vi "IMAQdx_AbsImage_Flea3_v4.6.vi"() -> ()   [LabVIEW 2013] (continued)
rMOTcurrF\trMOTpow3\tcombAmplitude(combWidthF)\trMOTdelta(-(rMOTbroadDetuningF +combWidthF/2))\tODTpowHLat(DipPowHLat2)\t0\t0\t0\t0\t0\t0\t1\t1\tbMOTdelta(MOTdetuning)\tbMOTpow(0.5)\tProbePow\tPdet2\tXshim\tYshim\tZshimVar\tODTpowZ(DipPowZLat)\t0\t1\t0\t0\t1\t0\t0\t0\t0\t0\t0\t0\t0\t0\t0\t0\t0\t0\trMOTdelta(-(rMOTstirDetI +stirWidthF/2))\tODTpowBlue(0)\tExpFinal(tEvap1,ODTpowXY(DipPowCr2),ODTpowXY(DipPowCr3),tau)\tvarWaveP2\tPdet\tAmp688(depumpPow)\trMOTpow3\tExpFinal(tEvap1,ODTpowX(DipPowX2),ODTpowX(DipPowX3),tau)\tfreq\tHeatingAmp\t0\tSine\tDetuning\tsingleFreqDet\tDoppCoolDet-DoppCoolSweep\tdopCoolT*1000\tDetuning\tsingleFreqStirDet + 20\tsingleFreqStirDet + 20\tSFcoolT*1000\tBlueBN\tBlueLaserProbeBN\tPixisPos(TOF)\tCycle Wait for Move\r\nlattice rampdown\t\tRamp\t0\trampLatOffT\t1\t1\t1\t1\t1\t1\t0\t0\t1\t1\t0\t0\t0\t1\t0\t0\t0\t1\t0\t0\t0\t0\t0\t0\t10u\t0\t1\t0\t0\t0\t1\t1\t0\tplus_zman\tminus_zman\tcompensation\trMOTcurrF\trMOTpow3\tcombAmplitude(combWidthF)\trMOTdelta(-(rMOTbroadDetuningF +combWidthF/2))\tSinRamp(t,(ODTpowHLat(DipPowHLat)+ODTpowHLat(DipPowHLat2))/2,(ODTpowHLat(DipPowHLat)-ODTpowHLat(DipPowHLat2))/2,1/(2*rampLatOffT), 3*pi/2)\t0\t0\t0\t0\t0\t0\t1\t1\tbMOTdelta(MOTdetuning)\tbMOTpow(0.5)\tProbePow\tPdet2\tXshim\tYshim\tZshimVar\tSinRamp(t,(ODTpowZ(DipPowZ3)+ODTpowZ(DipPowZLat))/2, (ODTpowZ(DipPowZ3)-ODTpowZ(DipPowZLat))/2, 1/(2*rampLatOffT), 3*pi/2)\t0\t1\t0\t0\t1\t0\t0\t0\t0\t0\t0\t0\t0\t0\t0\t0\t0\t0\trMOTdelta(-(rMOTstirDetI +stirWidthF/2))\tODTpowBlue(0)\tExpFinal(tEvap1,ODTpowXY(DipPowCr2),ODTpowXY(DipPowCr3),tau)\tLineRamp(f,varWaveP2,varWaveP1)\tPdet\tAmp688(depumpPow)\trMOTpow3\tExpFinal(tEvap1,ODTpowX(DipPowX2),ODTpowX(DipPowX3),tau)\tfreq\tHeatingAmp\t0\tSine\tDetuning\tsingleFreqDet\tDoppCoolDet-DoppCoolSweep\tdopCoolT*1000\tDetuning\tsingleFreqStirDet + 20\tsingleFreqStirDet + 20\tSFcoolT*1000\tBlueBN\tBlueLaserProbeBN\tPixisPos(TOF)\tCycle Wait for Move\r\nEvaporation\t\tRamp\t0\ttEvap2\t1\t1\t1\t1\t1\t1\t0\t0\t1\t1\t0\t0\t0\t1\t0\t0\t0\t1\t0\t0\t0\t0\t0\t0\t50u\t0\t1\t0\t0\t0\t1\t1\t0\tplus_zman\tminus_zman\tcompensation\trMOTcurrF\trMOTpow3\tcombAmplitude(combWidthF)\trMOTdelta(-(rMOTbroadDetuningF +combWidthF/2))\tODTpowHLat(DipPowHLat)\t0\t0\t0\t0\t0\t0\t1\t1\tbMOTdelta(MOTdetuning)\tbMOTpow(0.5)\tProbePow\tPdet2\tXshim\tYshim\tZshimVar\tLineRamp(f,ODTpowZ(DipPowZ3),ODTpowZ(DipPowZ4))\t0\t1\t0\t0\t0\t0\t0\t0\t0\t0\t0\t0\t0\t0\t0\t0\t0\t0\trMOTdelta(-(rMOTstirDetI +stirWidthF/2))\tODTpowBlue(0)\tExpRamp2(t,0,ExpFinal(tEvap1,ODTpowXY(DipPowCr2),ODTpowXY(DipPowCr3),tau),ODTpowXY(DipPowCr4),tau2)\tvarWaveP2\tPdet\tAmp688(depumpPow)\trMOTpow3\tExpRamp2(t,0,ExpFinal(tEvap1,ODTpowX(DipPowX2),ODTpowX(DipPowX3),tau),ODTpowX(DipPowX4),tau2)\tfreq\tHeatingAmp\t0\tSine\tDetuning\tsingleFreqDet\tDoppCoolDet-DoppCoolSweep\tdopCoolT*1000\tDetuning\tsingleFreqStirDet + 20\tsingleFreqStirDet + 20\tSFcoolT*1000\tBlueBN\tBlueLaserProbeBN\tPixisPos(TOF)\tCycle Wait for Move\r\npost evap hold\t\tRamp\t0\t.0075\t1\t1\t1\t1\t1\t1\t0\t0\t1\t1\t0\t0\t0\t1\t0\t0\t0\t1\t0\t0\t0\t0\t0\t0\t0\t0\t1\t0\t0\t0\t1\t1\t0\tplus_zman\tminus_zman\tcompensation\trMOTcurrF\trMOTpow3\tcombAmplitude(combWidthF)\trMOTdelta(-(rMOTbroadDetuningF +combWidthF/2))\tODTpowHLat(DipPowHLat)\t0\t0\t0\t0\t0\t0\t1\t1\tbMOTdelta(MOTdetuning)\tbMOTpow(0.5)\tProbePow\tPdet2\tXshim\tYshim\tZshimVar\tExpFinal(tEvap1,ODTpowZ(DipPowZ),ODTpowZ(DipPowZ2),tau)\tVimaging\t1\t0\t0\t0\t0\t0\t0\t0\t0\t0\t0\t0\t0\t0\t0\t0\t0\trMOTdelta(-(rMOTstirDetI +stirWidthF/2))\tODTpowBlue(0)\tExpFinal(tEvap1,ODTpowXY(DipPowCr),ODTpowXY(DipPowCr2),tau)\tvarWaveP2\tPdet\tAmp688(depumpPow)\trMOTpow3\tExpFinal(tEvap1,ODTpowX(DipPowX),ODTpowX(DipPowX2),tau)\tfreq\tHeatingAmp\t0\tSine\tDetuning\tsingleFreqDet\tDoppCoolDet-DoppCoolSweep\tdopCoolT*1000\tDetuning\tsingleFreqStirDet + 20\tsingleFreqStirDet + 20\tSFcoolT*1000\tBlueBN\tBlueLaserProbeBN\tPixisPos(TOF)\tCycle Wait for Move\r\nrMOT/Dip TOF\t\tRamp\t1\tTOFaux\t0\t0\t0\t0\t0\t0\t1\t0\t0\t1\t0\t0\t0\t0\t0\t0\t0\t1\t0\t0\t0\t0\t0\t0\t0\t0\t1\t0\t0\t0\t1\t1\t0\tplus_zman\tminus_zman\tcompensation\trMOTcurrF\trMOTpow5\tcombAmplitude(combWidthF)\trMOTdelta(-(rMOTbroadDetuningF +combWidthF/2))\tODTpowHLat(DipPowHLat2)\t0\tVimaging\t0\t0\t0\t1\t1\t1\tbMOTdelta(MOTdetuning)\tbMOTpow(0.5)\tProbePow\tPdet\tXshim\tYshim\tZshimVar\tODTpowZ(DipPowZ3)\tVimaging\t1\t0\tHimaging\t0\t0\t0\t0\t0\t0\t0\t0\t0\t0\t0\t0\t0\t0\trMOTdelta(-(rMOTstirDetI +stirWidthF/2))\tODTpowBlue(0)\tODTpowXY(DipPowCrTOF)\tvarWaveP2\tPdet\tAmp688(depumpPow)\trMOTpow6\tODTpowX(DipPowXTOF)\tfreq\tHeatingAmp\t0\tSine\tDetuning\tsingleFreqDetF\tDoppCoolDet-DoppCoolSweep\tdopCoolT*1000\tDetuning\tsingleFreqStirDet + 20\tsingleFreqStirDet + 20\tSFcoolT*1000\tBlueBN\tBlueLaserProbeBN\tPixisPos(TOF)\tCycle Wait for Move\r\nBEC in situ\t\tRamp\t0\tTOFaux\t1\t1\t1\t1\t1\t1\t1\t0\t0\t1\t0\t0\t0\t0\t0\t0\t0\t1\t0\t0\t0\t0\t0\t0\t0\t0\t1\t0\t0\t0\t1\t1\t0\tplus_zman\tminus_zman\tcompensation\trMOTcurrF\trMOTpow5\tcombAmplitude(combWidthF)\trMOTdelta(-(rMOTbroadDetuningF +combWidthF/2))\tODTpowHLat(DipPowHLat)\t0\tVimaging\t0\t0\t0\t1\t1\t1\tbMOTdelta(MOTdetuning)\tbMOTpow(0.5)\tProbePow\tPdet\tXshim\tYshim\tZshimVar\tODTpowZ(DipPowZ3)\tVimaging\t1\t0\tHimaging\t0\t0\t0\t0\t0\t0\t0\t0\t0\t0\t0\t0\t0\t0\trMOTdelta(-(rMOTstirDetI +stirWidthF/2))\tODTpowBlue(BlueDipPow)\tExpFinal(tEvap1,ODTpowXY(DipPowCr2),ODTpowXY(DipPowCr3),tau)\tvarWaveP1\tPdet\tAmp688(depumpPow)\trMOTpow6\tExpFinal(tEvap1,ODTpowX(DipPowX2),ODTpowX(DipPowX3),tau)\tfreq\tHeatingAmp\t0\tSine\tDetuning\tsingleFreqDetF\tDoppCoolDet-DoppCoolSweep\tdopCoolT*1000\tDetuning\tsingleFreqStirDet + 20\tsingleFreqStirDet + 20\tSFcoolT*1000\tBlueBN\tBlueLaserProbeBN\tPixisPos(TOF)\tCycle Wait for Move\r\nTOF\t\tRamp\t0\t.005\t0\t0\t0\t0\t0\t0\t1\t0\t0\t0\t0\t0\t0\t0\t0\t0\t0\t1\t0\t0\t0\t0\t0\t0\t0\t0\t1\t0\t0\t0\t1\t1\t0\tplus_zman\tminus_zman\tcompensation\trMOTcurrF\trMOTpow3\tcombAmplitude(combWidthF)\trMOTdelta(-(rMOTbroadDetuningF +combWidthF/2))\tODTpowHLat(DipPowHLat)\t1\tVimaging\t0\t0\t0\t1\t1\t1\tbMOTdelta(MOTdetuning)\tbMOTpow(0.5)\tProbePow\tPdet\tXshim\tYshim\tZshimVar\tODTpowZ(DipPowZ)\tVimaging\t1\t0\tHimaging\t0\t0\t0\t0\t0\t0\t0\t0\t0\t0\t0\t0\t0\t0\trMOTdelta(-(rMOTstirDetI +stirWidthF/2))\tODTpowBlue(0)\tODTpowXY(DipPowCr)\tvarWaveP2\tPdet\tAmp688(depumpPow)\trMOTpow3\tODTpowX(DipPowX2)\tfreq\tHeatingAmp\t0\tSine\tDetuning\tsingleFreqDet\tDoppCoolDet-DoppCoolSweep\tdopCoolT*1000\tDetuning\tsingleFreqStirDet\tsingleFreqStirDet + 20\tSFcoolT*1000\tBlueBN\tBlueLaserProbeBN\tPixisPos(TOF)\tCycle Wait for Move\r\nTOF\t\tRamp\t1-rMOTon\t.001\t0\t0\t0\t0\t0\t0\t1\t0\t0\t0\t0\t0\t0\t0\t0\t0\t0\t1\t0\t0\t0\t0\t0\t0\t0\t0\t1\t0\t0\t0\t1\t1\t0\tplus_zman\tminus_zman\tcompensation\trMOTcurrF\trMOTpow3\tcombAmplitude(combWidthF)\trMOTdelta(-(rMOTbroadDetuningF +combWidthF/2))\tODTpowHLat(DipPowHLat)\t1\tVimaging\t0\t0\t0\t1\t1\t1\tbMOTdelta(MOTdetuning)\tbMOTpow(0.5)\tProbePow\tPdet\tXshim\tYshim\tZshimVar\tODTpowZ(DipPowZ)\tVimaging\t1\t0\tHimaging\t0\t0\t0\t0\t0\t0\t0\t0\t0\t0\t0\t0\t0\t0\trMOTdelta(-(rMOTstirDetI +stirWidthF/2))\tODTpowBlue(0)\tODTpowXY(DipPowCr)\tvarWaveP2\tPdet\tAmp688(depumpPow)\trMOTpow3\tODTpowX(DipPowX2)\tfreq\tHeatingAmp\t0\tSine\tDetuning\tsingleFreqDet\tDoppCoolDet-DoppCoolSweep\tdopCoolT*1000\tDetuning\tsingleFreqStirDet\tsingleFreqStirDet + 20\tSFcoolT*1000\tBlueBN\tBlueLaserProbeBN\tPixisPos(TOF)\tCycle Wait for Move\r\narm DIP FLEA\t\tRamp\t1\tcameraArmT\t0\t0\t0\t0\t0\t0\t1\t0\t0\t0\t0\t0\t0\t0\t0\t0\t0\t0\t0\t0\t0\t0\t0\t0\t0\t0\t1\t0\t0\t0\t1\t0\t0\tplus_zman\tminus_zman\tcompensation\trMOTcurrF\trMOTpow3\tcombAmplitude(combWidthF)\trMOTdelta(-(rMOTbroadDetuningF +combWidthF/2))\tODTpowHLat(DipPowHLat)\t1\tVimaging\t0\t0\t0\t1\t1\t0\tbMOTdelta(MOTdetuning)\tbMOTpow(0.5)\tProbePow\tPdet\tXshim\tYshim\tZshimVar\tODTpowZ(DipPowZ3)\tVimaging\t1\t0\tHimaging\t0\t0\t0\t0\t0\t0\t0\t0\t0\t0\t0\t0\t0\t0\trMOTdelta(-(rMOTstirDetI +stirWidthF/2))\tODTpowBlue(0)\tODTpowXY(DipPowCrTOF)\tvarWaveP1\tPdet\tAmp688(depumpPow)\trMOTpow3\tODTpowX(DipPowXTOF)\tfreq\tHeatingAmp\t0\tSine\tDetuning\tsingleFreqDet\tDoppCoolDet-DoppCoolSweep\tdopCoolT*1000\tDetuning\tsingleFreqStirDet\tsingleFreqStirDet + 20\tSFcoolT*1000\tBlueBN\tBlueLaserProbeBN\tPixisPos(TOF)\tCycle Wait for Move\r\narm BEC FLEA\t\tRamp\t0\tcameraArmT\t0\t0\t0\t0\t0\t0\t1\t0\t0\t0\t0\t0\t0\t0\t0\t0\t0\t0\t0\t0\t0\t0\t0\t0\t0\t0\t1\t0\t0\t0\t1\t0\t0\tplus_zman\tminus_zman\tcompensation\trMOTcurrF\trMOTpow3\tcombAmplitude(combWidthF)\trMOTdelta(-(rMOTbroadDetuningF +combWidthF/2))\tODTpowHLat(DipPowHLat)\t1\tVimaging\t0\t0\t0\t1\t1\t0\tbMOTdelta(MOTdetuning)\tbMOTpow(0.5)\tProbePow\tPdet\tXshim\tYshim\tZshimVar\tODTpowZ(DipPowZ3)\tVimaging\t1\t0\tHimaging\t0\t0\t0\t0\t0\t0\t0\t0\t0\t0\t0\t0\t0\t0\trMOTdelta(-(rMOTstirDetI +stirWidthF/2))\tODTpowBlue(BlueDipPow)\tExpFinal(tEvap1,ODTpowXY(DipPowCr2),ODTpowXY(DipPowCr3),tau)\tvarWaveP1\tPdet\tAmp688(depumpPow)\trMOTpow3\tExpFinal(tEvap1,ODTpowX(DipPowX2),ODTpowX(DipPowX3),tau)\tfreq\tHeatingAmp\t0\tSine\tDetuning\tsingleFreqDet\tDoppCoolDet-DoppCoolSweep\tdopCoolT*1000\tDetuning\tsingleFreqStirDet\tsingleFreqStirDet + 20\tSFcoolT*1000\tBlueBN\tBlueLaserProbeBN\tPixisPos(TOF)\tCycle Wait for Move\r\natom img\t\tRamp\t1\texposureT\t0\t0\t0\t0\t0\t0\t1\t0\t1\t0\t0\t0\t0\t1\t0\t0\t0\t0\t0\t0\t0\t0\t0\t0\t0\t0\t1\t0\t0\t0\t1\t0\t0\tplus_zman\tminus_zman\tcompensation\trMOTcurrF\trMOTpow3\tcombAmplitude(combWidthF)\trMOTdelta(-(rMOTbroadDetuningF +combWidthF/2))\tODTpowHLat(DipPowHLat)\t1\tVimaging\t0\t0\t0\t1\t0\t0\tbMOTdelta(MOTdetuning)\tbMOTpow(0.5)\tProbePow\tPdet\tXshim\tYshim\tZshimVar\tODTpowZ(DipPowZ)\tVimaging\t1\t0\tHimaging\t0\t0\t0\t0\t0\t0\t0\t0\t0\t0\t0\t0\t0\t0\trMOTdelta(-(rMOTstirDetI +stirWidthF/2))\tODTpowBlue(0)\tODTpowXY(DipPowCr)\tvarWaveP1\tPdet\tAmp688(depumpPow)\trMOTpow3\tODTpowX(DipPowX)\tfreq\tHeatingAmp\t0\tSine\tDetuning\tsingleFreqDet\tDoppCoolDet-DoppCoolSweep\tdopCoolT*1000\tDetuning\tsingleFreqStirDet\tsingleFreqStirDet + 20\tSFcoolT*1000\tBlueBN\tBlueLaserProbeBN\tPixisPos(TOF)\tCycle Wait for Move\r\natom img\t\tRamp\t0\t2.8e-3\t0\t0\t0\t0\t0\t0\t1\t0\t0\t1\t0\t0\t0\t0\t0\t0\t0\t0\t0\t0\t0\t0\t0\t0\t0\t0\t1\t0\t0\t0\t1\t1\t0\tplus_zman\tminus_zman\tcompensation\trMOTcurrF\trMOTpow3\tcombAmplitude(combWidthF)\trMOTdelta(-(rMOTbroadDetuningF +combWidthF/2))\tODTpowHLat(DipPowHLat)\t1\tVimaging\t0\t0\t0\t1\t1\t1\tbMOTdelta(MOTdetuning)\tbMOTpow(0.5)\tProbePow\tPdet\tXshim\tYshim\tZshimVar\tODTpowZ(DipPowZ)\tVimaging\t1\t0\tHimaging\t0\t0\t0\t0\t0\t0\t0\t0\t0\t0\t0\t0\t0\t0\trMOTdelta(-(rMOTstirDetI +stirWidthF/2))\tODTpowBlue(0)\tODTpowXY(DipPowCr)\tvarWaveP2\tPdet\tAmp688(depumpPow)\trMOTpow3\tODTpowX(DipPowX)\tfreq\tHeatingAmp\t0\tSine\tDetuning\tsingleFreqDet\tDoppCoolDet-DoppCoolSweep\tdopCoolT*1000\tDetuning\tsingleFreqStirDet\tsingleFreqStirDet + 20\tSFcoolT*1000\tBlueBN\tBlueLaserProbeBN\tPixisPos(TOF)\tCycle Wait for Move\r\ntransmit img\t\tRamp\t1\t.625\t0\t0\t0\t0\t0\t0\t1\t0\t0\t1\t0\t0\t0\t0\t0\t0\t0\t0\t0\t0\t0\t0\t0\t0\t0\t0\t1\t0\t0\t0\t1\t1\t0\tplus_zman\tminus_zman\tcompensation\trMOTcurrF\trMOTpow3\tcombAmplitude(combWidthF)\trMOTdelta(-(rMOTbroadDetuningF +combWidthF/2))\tODTpowHLat(DipPowHLat)\t1\tVimaging\t0\t0\t0\t1\t1\t1\tbMOTdelta(MOTdetuning)\tbMOTpow(0.5)\tProbePow\tPdet\tXshim\tYshim\tZshimVar\tODTpowZ(DipPowZ)\tVimaging\t1\t0\tHimaging\t0\t0\t0\t0\t0\t0\t0\t0\t0\t0\t0\t0\t0\t0\trMOTdelta(-(rMOTstirDetI +stirWidthF/2))\tODTpowBlue(0)\tODTpowXY(DipPowCr)\tvarWaveP2\tPdet\tAmp688(depumpPow)\trMOTpow3\tODTpowX(DipPowX)\tfreq\tHeatingAmp\t0\tSine\tDetuning\tsingleFreqDet\tDoppCoolDet-DoppCoolSweep\tdopCoolT*1000\tDetuning\tsingleFreqStirDet\tsingleFreqStirDet + 20\tSFcoolT*1000\tBlueBN\tBlueLaserProbeBN\tPixisPos(TOF)\tCycle Wait for Move\r\narm PIXIS\t\tRamp\t0\t.007\t0\t0\t0\t0\t0\t0\t1\t0\t0\t1\t1\t0\t0\t0\t1\t1\t0\t0\t0\t0\t0\t0\t0\t0\t0\t0\t1\t0\t0\t0\t1\t1\t0\tplus_zman\tminus_zman\tcompensation\trMOTcurrF\trMOTpow1\tcombAmplitude(combWidthF)\trMOTdelta(-(rMOTbroadDetuningF +combWidthF/2))\tODTpowHLat(DipPowHLat)\t1\tVimaging\t0\t0\t0\t1\t1\t1\tbMOTdelta(MOTdetuning)\tbMOTpow(0.5)\tProbePow\tPdet\tXshim\tYshim\tZshimVar\tODTpowZ(DipPowZ)\tVimaging\t1\t0\tHimaging\t0\t0\t0\t0\t0\t0\t0\t0\t0\t0\t0\t0\t0\t0\trMOTdelta(-(rMOTstirDetI +stirWidthF/2))\tODTpowBlue(0)\tODTpowXY(DipPowCr)\tvarWaveP2\tPdet\tAmp688(depumpPow)\trMOTpow1\tODTpowX(DipPowX)\tfreq\tHeatingAmp\t0\tSine\tDetuning\tsingleFreqDet\tDoppCoolDet-DoppCoolSweep\tdopCoolT*1000\tDetuning\tsingleFreqStirDet\tsingleFreqStirDet + 20\tSFcoolT*1000\tBlueBN\tBlueLaserProbeBN\tPixisPos(TOF)\tCycle Wait for Move\r\narm FLEA\t\tRamp\t1\tcameraArmT\t0\t0\t0\t0\t0\t0\t1\t0\t0\t1\t1\t0\t0\t0\t1\t1\t0\t0\t0\t0\t0\t0\t0\t0\t0\t0\t1\t0\t0\t0\t1\t0\t0\tplus_zman\tminus_zman\tcompensation\trMOTcurrF\trMOTpow1\tcombAmplitude(combWidthF)\trMOTdelta(-(rMOTbroadDetuningF +combWidthF/2))\tODTpowHLat(DipPowHLat)\t1\tVimaging\t0\t0\t0\t1\t1\t0\tbMOTdelta(MOTdetuning)\tbMOTpow(0.5)\tProbePow\tPdet\tXshim\tYshim\tZshimVar\tODTpowZ(DipPowZ)\tVimaging\t1\t0\tHimaging\t0\t0\t0\t0\t0\t0\t0\t0\t0\t0\t0\t0\t0\t0\trMOTdelta(-(rMOTstirDetI +stirWidthF/2))\tODTpowBlue(0)\tODTpowXY(DipPowCr)\tvarWaveP2\tPdet\tAmp688(depumpPow)\trMOTpow1\tODTpowX(DipPowX)\tfreq\tHeatingAmp\t0\tSine\tDetuning\tsingleFreqDet\tDoppCoolDet-DoppCoolSweep\tdopCoolT*1000\tDetuning\tsingleFreqStirDet\tsingleFreqStirDet + 20\tSFcoolT*1000\tBlueBN\tBlueLaserProbeBN\tPixisPos(TOF)\tCycle Wait for Move\r\nprobe img\t\tRamp\t1\texposureT\t0\t0\t0\t0\t0\t0\t1\t0\t1\t1\t1\t0\t0\t1\t1\t1\t0\t0\t0\t0\t0\t0\t0\t0\t0\t0\t1\t0\t0\t0\t1\t0\t0\tplus_zman\tminus_zman\tcompensation\trMOTcurrF\trMOTpow1\tcombAmplitude(combWidthF)\trMOTdelta(-(rMOTbroadDetuningF +combWidthF/2))\tODTpowHLat(DipPowHLat)\t1\tVimaging\t0\t0\t0\t1\t0\t0\tbMOTdelta(MOTdetuning)\tbMOTpow(0.5)\tProbePow\tPdet\tXshim\tYshim\tZshimVar\tODTpowZ(DipPowZ)\tVimaging\t1\t0\tHimaging\t0\t0\t0\t0\t0\t0\t0\t0\t0\t0\t0\t0\t0\t0\trMOTdelta(-(rMOTstirDetI +stirWidthF/2))\tODTpowBlue(0)\tODTpowXY(DipPowCr)\tvarWaveP2\tPdet\tAmp688(depumpPow)\trMOTpow1\tODTpowX(DipPowX)\tfreq\tHeatingAmp\t0\tSine\tDetuning\tsingleFreqDet\tDoppCoolDet-DoppCoolSweep\tdopCoolT*1000\tDetuning\tsingleFreqStirDet\tsingleFreqStirDet + 20\tSFcoolT*1000\tBlueBN\tBlueLaserProbeBN\tPixisPos(TOF)\tCycle Wait for Move\r\nprobe img\t\tRamp\t0\t2.8e-3\t0\t0\t0\t0\t0\t0\t1\t0\t0\t1\t1\t0\t0\t0\t1\t1\t0\t0\t0\t0\t0\t0\t0\t0\t0\t0\t1\t0\t0\t0\t1\t1\t0\tplus_zman\tminus_zman\tcompensation\trMOTcurrF\trMOTpow1\tcombAmplitude(combWidthF)\trMOTdelta(-(rMOTbroadDetuningF +combWidthF/2))\tODTpowHLat(DipPowHLat)\t1\tVimaging\t0\t0\t0\t1\t1\t1\tbMOTdelta(MOTdetuning)\tbMOTpow(0.5)\tProbePow\tPdet\tXshim\tYshim\tZshimVar\tODTpowZ(DipPowZ)\tVimaging\t1\t0\tHimaging\t0\t0\t0\t0\t0\t0\t0\t0\t0\t0\t0\t0\t0\t0\trMOTdelta(-(rMOTstirDetI +stirWidthF/2))\tODTpowBlue(0)\tODTpowXY(DipPowCr)\tvarWaveP2\tPdet\tAmp688(depumpPow)\trMOTpow1\tODTpowX(DipPowX)\tfreq\tHeatingAmp\t0\tSine\tDetuning\tsingleFreqDet\tDoppCoolDet-DoppCoolSweep\tdopCoolT*1000\tDetuning\tsingleFreqStirDet\tsingleFreqStirDet + 20\tSFcoolT*1000\tBlueBN\tBlueLaserProbeBN\tPixisPos(TOF)\tCycle Wait for Move\r\ntransmit img\t\tRamp\t1\t.610\t0\t0\t0\t0\t0\t0\t1\t0\t0\t1\t1\t0\t0\t0\t1\t1\t0\t0\t0\t0\t0\t0\t0\t0\t0\t0\t1\t0\t0\t0\t1\t1\t0\tplus_zman\tminus_zman\tcompensation\trMOTcurrF\trMOTpow1\tcombAmplitude(combWidthF)\trMOTdelta(-(rMOTbroadDetuningF +combWidthF/2))\tODTpowHLat(DipPowHLat)\t1\tVimaging\t0\t0\t0\t1\t1\t1\tbMOTdelta(MOTdetuning)\tbMOTpow(0.5)\tProbePow\tPdet\tXshim\tYshim\tZshimVar\tODTpowZ(DipPowZ)\tVimaging\t1\t0\tHimaging\t0\t0\t0\t0\t0\t0\t0\t0\t0\t0\t0\t0\t0\t0\trMOTdelta(-(rMOTstirDetI +stirWidthF/2))\tODTpowBlue(0)\tODTpowXY(DipPowCr)\tvarWaveP2\tPdet\tAmp688(depumpPow)\trMOTpow1\tODTpowX(DipPowX)\tfreq\tHeatingAmp\t0\tSine\tDetuning\tsingleFreqDet\tDoppCoolDet-DoppCoolSweep\tdopCoolT*1000\tDetuning\tsingleFreqStirDet\tsingleFreqStirDet + 20\tSFcoolT*1000\tBlueBN\tBlueLaserProbeBN\tPixisPos(TOF)\tCycle Wait for Move\r\ntransmit img\t\tRamp\t1\t.015\t0\t0\t0\t0\t0\t0\t1\t0\t0\t1\t1\t0\t0\t0\t1\t1\t0\t0\t0\t0\t0\t0\t0\t0\t0\t0\t1\t0\t0\t0\t1\t1\t0\tplus_zman\tminus_zman\tcompensation\trMOTcurrF\trMOTpow1\tcombAmplitude(combWidthF)\trMOTdelta(-(rMOTbroadDetuningF +combWidthF/2))\tODTpowHLat(DipPowHLat2)\t1\tVimaging\t0\t0\t0\t1\t1\t1\tbMOTdelta(MOTdetuning)\tbMOTpow(0.5)\tProbePow\tPdet\tXshim\tYshim\tZshimVar\tODTpowZ(DipPowZ)\tVimaging\t1\t0\tHimaging\t0\t0\t0\t0\t0\t0\t0\t0\t0\t0\t0\t0\t0\t0\trMOTdelta(-(rMOTstirDetI +stirWidthF/2))\tODTpowBlue(.05)\tODTpowXY(DipPowCr)\tvarWaveP2\tPdet\tAmp688(depumpPow)\trMOTpow1\tODTpowX(DipPowX)\tfreq\tHeatingAmp\t0\tSine\tDetuning\tsingleFreqDet\tDoppCoolDet-DoppCoolSweep\tdopCoolT*1000\tDetuning\tsingleFreqStirDet\tsingleFreqStirDet + 20\tSFcoolT*1000\tBlueBN\tBlueLaserProbeBN\tPixisPos(TOF)\tCycle Wait for Move\r\narm PIXIS\t\tRamp\t0\t.007\t0\t0\t0\t0\t0\t0\t1\t0\t0\t1\t1\t0\t0\t0\t1\t1\t0\t0\t0\t0\t0\t0\t0\t0\t0\t0\t1\t0\t0\t0\t1\t0\t0\tplus_zman\tminus_zman\tcompensation\trMOTcurrF\trMOTpow1\tcombAmplitude(combWidthF)\trMOTdelta(-(rMOTbroadDetuningF +combWidthF/2))\tODTpowHLat(DipPowHLat2)\t1\tVimaging\t0\t0\t0\t1\t1\t1\tbMOTdelta(MOTdetuning)\tbMOTpow(0.5)\tProbePow\tPdet\tXshim\tYshim\tZshimVar\tODTpowZ(DipPowZ)\tVimaging\t1\t0\tHimaging\t0\t0\t0\t0\t0\t0\t0\t0\t0\t0\t0\t0\t0\t0\trMOTdelta(-(rMOTstirDetI +stirWidthF/2))\tODTpowBlue(0)\tODTpowXY(DipPowCr)\tvarWaveP2\tPdet\tAmp688(depumpPow)\trMOTpow1\tODTpowX(DipPowX)\tfreq\tHeatingAmp\t0\tSine\tDetuning\tsingleFreqDet\tDoppCoolDet-DoppCoolSweep\tdopCoolT*1000\tDetuning\tsingleFreqStirDet\tsingleFreqStirDet + 20\tSFcoolT*1000\tBlueBN\tBlueLaserProbeBN\tPixisPos(TOF)\tCycle Wait for Move\r\narm FLEA\t\tRamp\t1\tcameraArmT\t0\t0\t0\t0\t0\t0\t1\t0\t0\t1\t1\t0\t0\t0\t1\t1\t0\t0\t0\t0\t0\t0\t0\t0\t0\t0\t1\t0\t0\t0\t1\t0\t0\tplus_zman\tminus_zman\tcompensation\trMOTcurrF\trMOTpow1\tcombAmplitude(combWidthF)\trMOTdelta(-(rMOTbroadDetuningF +combWidthF/2))\tODTpowHLat(DipPowHLat2)\t1\tVimaging\t0\t0\t0\t1\t1\t0\tbMOTdelta(MOTdetuning)\tbMOTpow(0.5)\tProbePow\tPdet\tXshim\tYshim\tZshimVar\tODTpowZ(DipPowZ)\tVimaging\t1\t0\tHimaging\t0\t0\t0\t0\t0\t0\t0\t0\t0\t0\t0\t0\t0\t0\trMOTdelta(-(rMOTstirDetI +stirWidthF/2))\tODTpowBlue(.05)\tODTpowXY(DipPowCr)\tvarWaveP2\tPdet\tAmp688(depumpPow)\trMOTpow1\tODTpowX(DipPowX)\tfreq\tHeatingAmp\t0\tSine\tDetuning\tsingleFreqDet\tDoppCoolDet-DoppCoolSweep\tdopCoolT*1000\tDetuning\tsingleFreqStirDet\tsingleFreqStirDet + 20\tSFcoolT*1000\tBlueBN\tBlueLaserProbeBN\tPixisPos(TOF)\tCycle Wait for Move\r\nbg img\t\tRamp\t1\texposureT\t0\t0\t0\t0\t0\t0\t1\t0\t0\t1\t1\t0\t0\t0\t1\t1\t0\t0\t0\t0\t0\t0\t0\t0\t0\t0\t1\t0\t0\t0\t1\t0\t0\tplus_zman\tminus_zman\tcompensation\trMOTcurrF\trMOTpow1\tcombAmplitude(combWidthF)\trMOTdelta(-(rMOTbroadDetuningF +combWidthF/2))\tODTpowHLat(DipPowHLat2)\t1\tVimaging\t0\t0\t0\t1\t0\t0\tbMOTdelta(MOTdetuning)\tbMOTpow(0.5)\tProbePow\tPdet\tXshim\tYshim\tZshimVar\tODTpowZ(DipPowZ)\tVimaging\t1\t0\tHimaging\t0\t0\t0\t0\t0\t0\t0\t0\t0\t0\t0\t0\t0\t0\trMOTdelta(-(rMOTstirDetI +stirWidthF/2))\tODTpowBlue(0)\tODTpowXY(DipPowCr)\tvarWaveP2\tPdet\tAmp688(depumpPow)\trMOTpow1\tODTpowX(DipPowX)\tfreq\tHeatingAmp\t0\tSine\tDetuning\tsingleFreqDet\tDoppCoolDet-DoppCoolSweep\tdopCoolT*1000\tDetuning\tsingleFreqStirDet\tsingleFreqStirDet + 20\tSFcoolT*1000\tBlueBN\tBlueLaserProbeBN\tPixisPos(TOF)\tCycle Wait for Move\r\nbg img\t\tRamp\t0\t1e-4\t0\t0\t0\t0\t0\t0\t1\t0\t0\t1\t1\t0\t0\t0\t1\t1\t0\t0\t0\t0\t0\t0\t0\t0\t0\t0\t1\t0\t0\t0\t1\t1\t0\tplus_zman\tminus_zman\tcompensation\trMOTcurrF\trMOTpow1\tcombAmplitude(combWidthF)\trMOTdelta(-(rMOTbroadDetuningF +combWidthF/2))\tODTpowHLat(DipPowHLat)\t1\tVimaging\t0\t0\t0\t1\t1\t1\tbMOTdelta(MOTdetuning)\tbMOTpow(0.5)\tProbePow\tPdet\tXshim\tYshim\tZshimVar\tODTpowZ(DipPowZ)\tVimaging\t1\t0\tHimaging\t0\t0\t0\t0\t0\t0\t0\t0\t0\t0\t0\t0\t0\t0\trMOTdelta(-(rMOTstirDetI +stirWidthF/2))\tODTpowBlue(0)\tODTpowXY(DipPowCr)\tvarWaveP2\tPdet\tAmp688(depumpPow)\trMOTpow1\tODTpowX(DipPowX)\tfreq\tHeatingAmp\t0\tSine\tDetuning\tsingleFreqDet\tDoppCoolDet-DoppCoolSweep\tdopCoolT*1000\tDetuning\tsingleFreqStirDet\tsingleFreqStirDet + 20\tSFcoolT*1000\tBlueBN\tBlueLaserProbeBN\tPixisPos(TOF)\tCycle Wait for Move\r\ntransmit img\t\tRamp\t1\t.625\t0\t0\t0\t0\t0\t0\t1\t1\t0\t1\t1\t0\t0\t0\t1\t1\t0\t0\t0\t0\t0\t0\t0\t0\t0\t0\t1\t0\t0\t0\t1\t1\t0\tplus_zman\tminus_zman\tcompensation\trMOTcurrF\trMOTpow1\tcombAmplitude(combWidthF)\trMOTdelta(-(rMOTbroadDetuningF +combWidthF/2))\tODTpowHLat(DipPowHLat)\t1\tVimaging\t0\t0\t0\t1\t1\t1\tbMOTdelta(MOTdetuning)\tbMOTpow(0.5)\tProbePow\tLineRamp(f,Pdet,Pdet2)\tXshim\tYshim\tZshimVar\tODTpowZ(DipPowZ)\tVimaging\t1\t0\tHimaging\t0\t0\t0\t0\t0\t0\t0\t0\t0\t0\t0\t0\t0\t0\trMOTdelta(-(rMOTstirDetI +stirWidthF/2))\tODTpowBlue(0)\tODTpowXY(DipPowCr)\tvarWaveP2\tPdet\tAmp688(depumpPow)\trMOTpow1\tODTpowX(DipPowX)\tfreq\tHeatingAmp\t0\tSine\tDetuning\tsingleFreqDet\tDoppCoolDet-DoppCoolSweep\tdopCoolT*1000\tDetuning\tsingleFreqStirDet\tsingleFreqStirDet + 20\tSFcoolT*1000\tBlueBN\tBlueLaserProbeBN\tPixisPos(TOF)\tCycle Wait for Move\r\nalignment\t\tRamp\t1\t.1\t1\t1\t1\t1\t1\t1\t1\t0\t1\t0\t1\t0\t1\t1\t1\t1\t0\t0\t0\t0\t0\t0\t0\t0\t1m\t0\t1\t0\t1\t0\t0\t1\t1\tplus_zman\tminus_zman\tcompensation\tMOTcurrent\trMOTpow1\tcombAmplitude(combWidthI)\trMOTdelta(-(rMOTbroadDetuningI +combWidthI/2))\tODTpowHLat(DipPowHLat2)\t1\t0\t1\t1\t0\t1\t1\t1\tbMOTdelta(MOTdetuning)\tbMOTpow(MOTPow)\tProbePow\tPdet2\tXshim\tYshim\tZshim\tODTpowZ(DipPowZLat)\t0\t1\t0\t0\t0\t1\t0\t0\t0\t0\t0\t0\t0\t0\t0\t0\t0\t0\trMOTdelta(-(rMOTstirDetI +stirWidthI/2))\tODTpowBlue(0)\tODTpowXY(DipPowCr)\tvarWaveP2\tLineRamp(f,Pdet,BlueLaserLockOffset)\tAmp688(depumpPow)\trMOTpow3\tODTpowX(DipPowX)\tfreq\tHeatingAmp\t0\tSine\tRamp\tsingleFreqDet\tsingleFreqDetF\tSFcoolT*1000\tRamp\tsingleFreqStirDet\tsingleFreqStirDetF\tSFcoolT*1000\tBlueBN\tBlueLaserBeatnote\tPixisPos(TOF)\tCycle Wait for Move\r\n\r\n\r\n"
  in  "Flea Wave Name":string="Test_Img"
  in  "Save files to archive?":bool=TRUE
  out "Timeout":bool=TRUE
  out "Trigger Overrun":bool=TRUE
  in  "Source of File Data":refnum<k21>="\\\\Control\\VariableLibrary\\Instruction String"
  in  "Timeout (ms)":u32=20000
  in  "Gain":dbl
  in  "Shutter speed":dbl=30000.0
  in  "PIXIS Magnification":dbl=5.48
  in  "PIXIS Image direction":enum16{"XY", "XZ"}(ring)
  in  "PIXIS Imaging technique":enum16{"Absorption", "Fluorescence", "RawImage"}(ring)
  in  "SPE File Path":path=path "C:/Users/Lab/Documents/LightField/LabviewTemp.spe"
  in  "Send PIXIS data to Igor?":bool
  in  "PIXIS File Parameters":T1={"Data Root"=path "I:/Data", "Index"=4, "Instrument"="PIXIS"} {"Index" format="%04d"}
  in  "Source of Wavemeter Data":refnum<k21>="\\\\WS7PC\\VariableLibrary\\Frequency"
  in  "Accept wavelength from remote system":bool=TRUE
  in  "Flea Raw image to view":u16(ring)=1 items=["Clear", "Absorbtion", "Probe", "Background"]
  in  "Update Graphics":bool=TRUE
  out "Flea Raw Image":u16[][](graph)
  out "Flea Processed Image":sgl[][](graph)
  out "PIXIS Processed Image":sgl[][](graph)
  out "PIXIS Raw Image":u16[][](graph)
  in  "PIXIS Raw image to view":u16(ring)=1 items=["Clear", "Absorbtion", "Probe", "Background"]
  out "Camera Error":errorcluster={"status"=FALSE, "code"=-1074360293, "source"="IMAQdx Get Image2.vi"}
  out "DDE Error":errorcluster={"status"=FALSE, "code"=0, "source"="DDE Close: No Error"}
  out "Status Array":T4(array[cluster])=[{"AcquisitionInProgress"=FALSE, "BufferCount"=0, "LastBufferNumber"=4294967292, "LostBufferCount"=0}, {"AcquisitionInProgress"=TRUE, "BufferCount"=0, "LastBufferNumber"=4294967292, "LostBufferCount"=0}, {"AcquisitionInProgress"=TRUE, "BufferCount"=0, "LastBufferNumber"=4294967292, "LostBufferCount"=0}, {"AcquisitionInProgress"=TRUE, "BufferCount"=0, "LastBufferNumber"=4294967292, "LostBufferCount"=0}, {"AcquisitionInProgress"=TRUE, "BufferCount"=0, "LastBufferNumber"=4294967292, "LostBufferCount"=0}, {"AcquisitionInProgress"=TRUE, "BufferCount"=0, "LastBufferNumber"=4294967292, "LostBufferCount"=0}, {"AcquisitionInProgress"=TRUE, "BufferCount"=0, "LastBufferNumber"=4294967292, "LostBufferCount"=0}, {"AcquisitionInProgress"=TRUE, "BufferCount"=0, "LastBufferNumber"=4294967292, "LostBufferCount"=0}, {"AcquisitionInProgress"=TRUE, "BufferCount"=0, "LastBufferNumber"=4294967292, "LostBufferCount"=0}, {"AcquisitionInProgress"=TRUE, "BufferCount"=1, "LastBufferNumber"=0, "LostBufferCount"=0}, {"AcquisitionInProgress"=TRUE, "BufferCount"=2, "LastBufferNumber"=1, "LostBufferCount"=0}, {"AcquisitionInProgress"=TRUE, "BufferCount"=3, "LastBufferNumber"=2, "LostBufferCount"=0}, {"AcquisitionInProgress"=TRUE, "BufferCount"=4, "LastBufferNumber"=3, "LostBufferCount"=0}]
  in  "SPE Load Error In":errorcluster
  out "DataBlock Info":T5={"frame count"=4, "frame size"=524288, "frame stride"=524288, "N ROI"=1, "ROI widths"=[512], "ROI heights"=[512], "ROI sizes"=[524288], "ROI strides"=[524288]}
  out "DS Error":errorcluster
  out "XML Parse Errors":string
  out "Data Array Size":i32=1
  out "SPE Load Error Out":errorcluster
  out "Flea Path":path=path "I:/Data/2016/April/22/FL3_32S2M_22Apr2016_0160.ibw"
  out "PIXIS Path":path=path "C:/Experiment/Data/PIXIStemp.ibw"
  out "PIXIS Images":u16[][][](array[numeric])
  out "Flea Images":u16[][][](array[numeric])
  out "Buffer Number":u32=4294967294
  out "Flea Frames":i32
  out "Flea Loop":i32=16
  # "Image Acquisition v4.6 (FOR USB3 CAMERAS ONLY!!!)"
  # "Experimental Parameters"
  # "These are only get set on 1st run.\nUse a Gain of 0, Shutter Speed not used"
  # "In both techniques 3 images\nare aquired, but in Fluorescense\nthe 3rd is discarded"
  # "Sr: .663  is XZ a\n     .898 is XZ b\n      5.48 is XY"
  # "Obsolete: (now done with network variables)\nWhen paramaters are accepted from a remote system a DataSockets server\nmust be running on this machine (in start menu in National Instruments folder)"
  # "Camera configuration"
  # "File configuration"
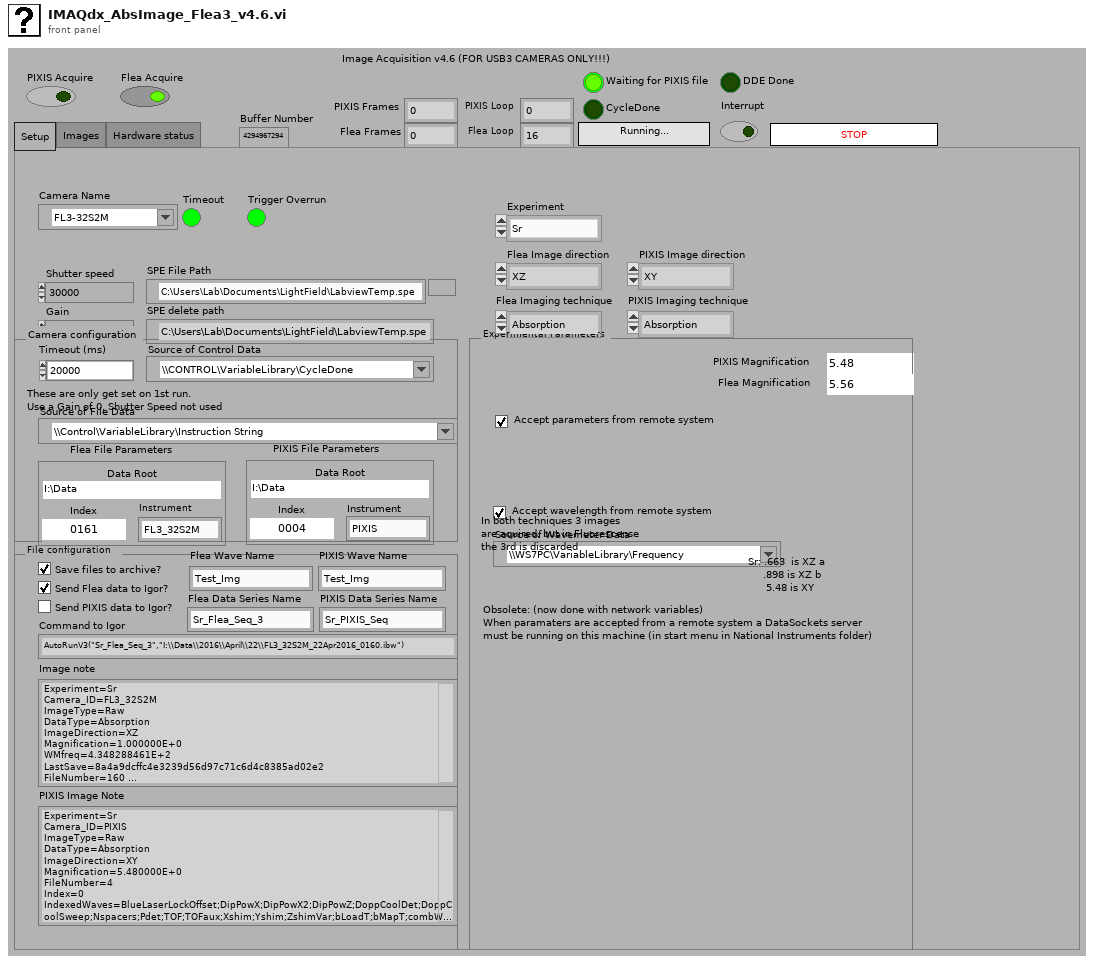
[diagram p1: front panel]
types:
  T1 = typedef "FileName_Cluster.ctl" = cluster{"Data Root":path, "Index":u32, "Instrument":string}
  T2 = typedef "IMAQdx.ctl" = refnum<k21>
  T3 = enum16{"Rubidium I", "Rubidium II", "RbLi", "RbYb", "Sr"}
  T4 = cluster{"AcquisitionInProgress":bool, "BufferCount":u32, "LastBufferNumber":u32, "LostBufferCount":u32}[]
  T5 = cluster{"frame count":i64, "frame size":i64, "frame stride":i64, "N ROI":i64, "ROI widths":i64[], "ROI heights":i64[], "ROI sizes":i64[], "ROI strides":i64[]}
  T6 = typedef "NI_Vision_Acquisition_Software.lvlib/IMAQdx Acquisition Mode.ctl" = enum32{"One Shot", "Continuous"}
  T7 = typedef "Image Type" = u32
  T8 = typedef "IMAQ Image.ctl" = refnum<image>
  T9 = cluster{"AcquisitionInProgress":bool, "BufferCount":u32, "LastBufferNumber":u32, "LostBufferCount":u32}
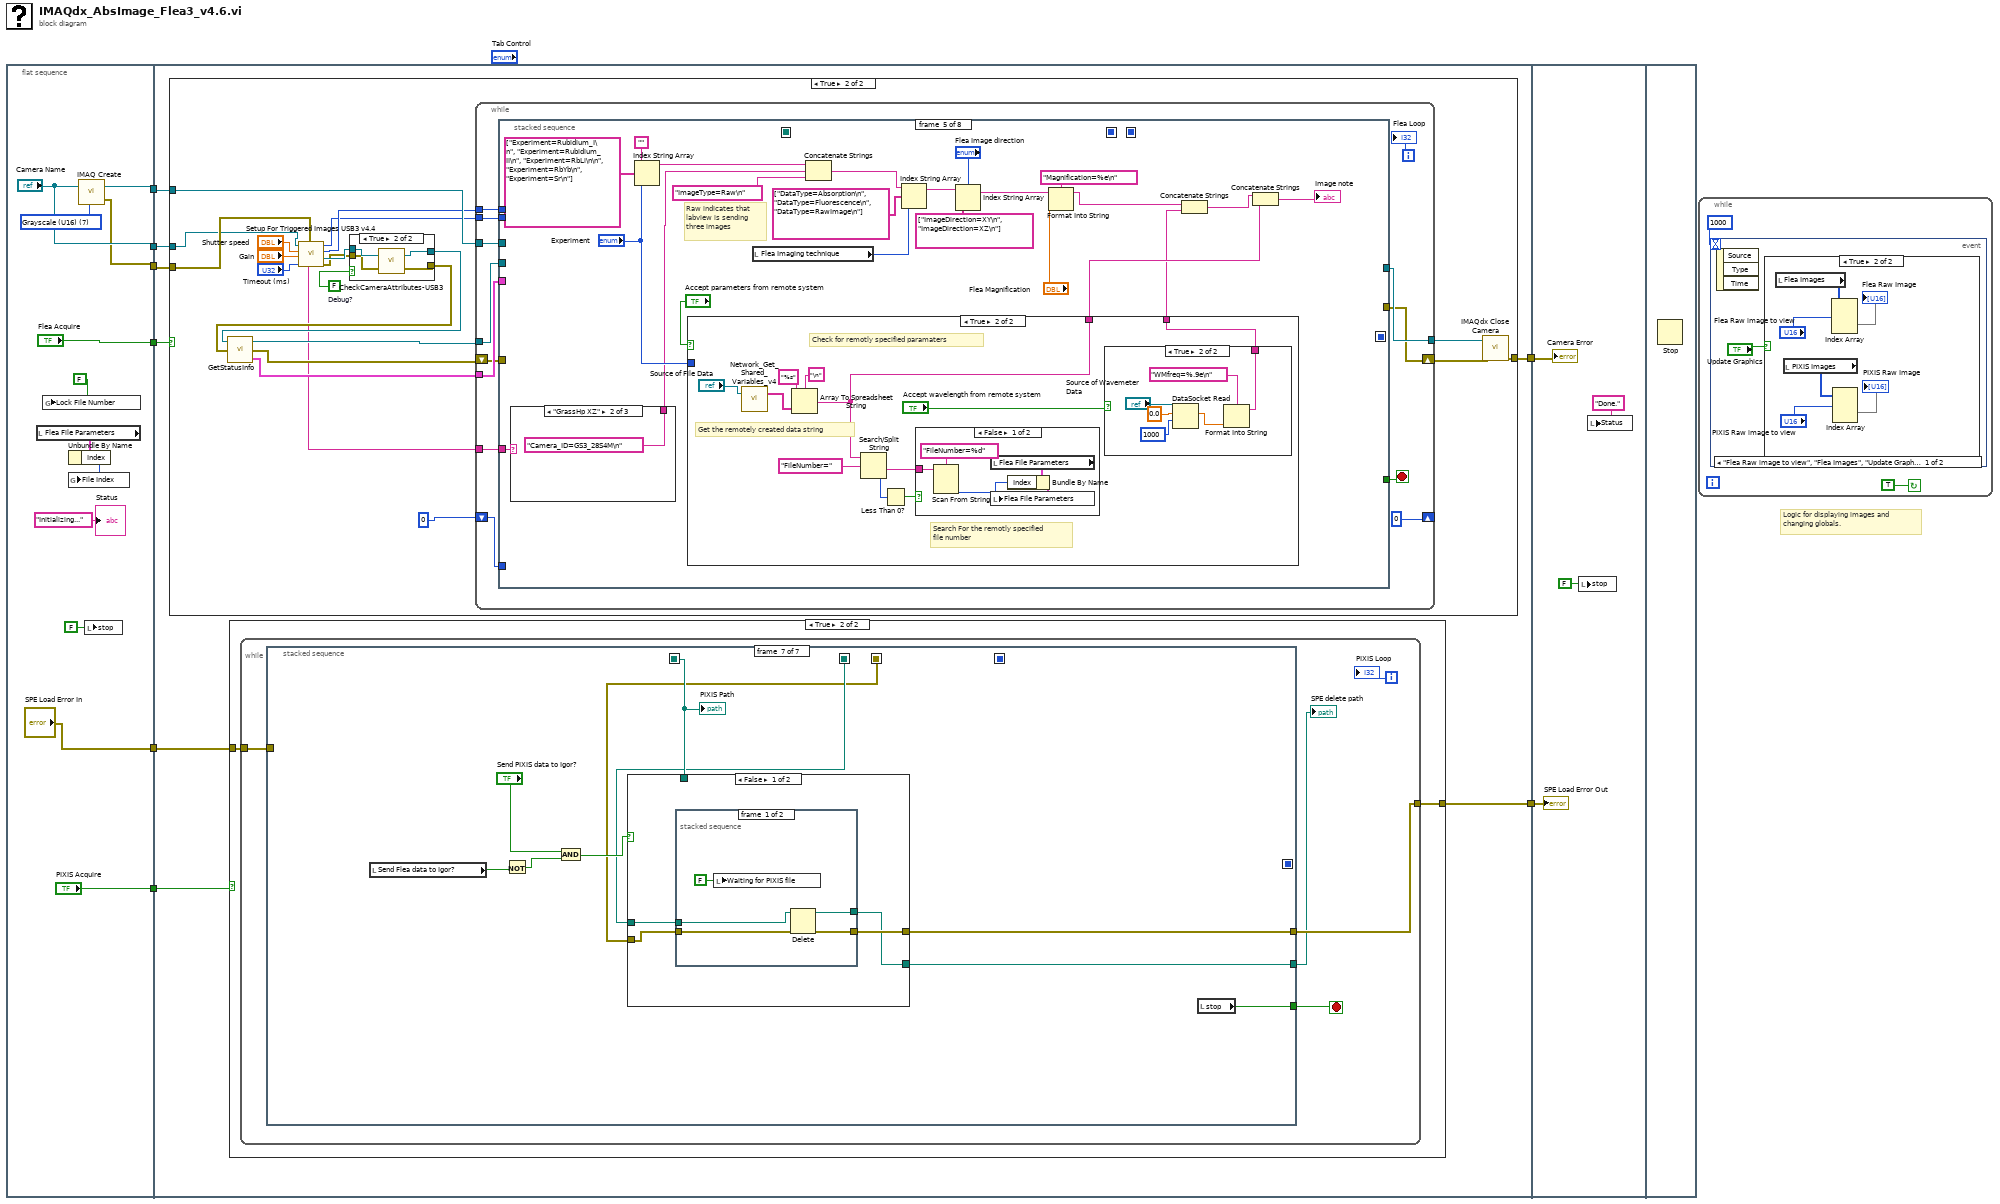
[diagram p0: block diagram]
diagram:
  # "Logic for displaying images and\nchanging globals."
  n1 = flat-sequence {
    tunnel: [w16] -> w8
    tunnel: ["Camera Name"] -> w7
    tunnel: [w14] -> w6
    tunnel: ["SPE Load Error In"] -> w5
    tunnel: ["PIXIS Acquire"] -> w3
    tunnel: ["Flea Acquire"] -> w1
    tunnel: w7 -> [w28]
    tunnel: w8 -> [w26]
    tunnel: w6 -> [w27]
    tunnel: w5 -> [w25]
    tunnel: [w24] -> w4
    tunnel: w3 -> [w23]
    tunnel: [w22] -> w2
    tunnel: w1 -> [w21]
    tunnel: w4 -> [w473]
    tunnel: w2 -> [w472]
    frame #0 {
      w13 = T7 7 items=["Grayscale (U8)", "Grayscale (I16)", "Grayscale (SGL)", "Complex (CSG)", "RGB (U32)", "HSL (U32)", "RGB (U64)", "Grayscale (U16)"] ("Image Type")
      n2 = local read "Flea File Parameters"() -> (w17:T1)
      n3 = global write "FileInfo_Global.vi" "Lock File Number"(FALSE) -> ()
      n4 = Unbundle By Name(w17) -> ("Index"=w18:u32)
      n5 = global write "FileInfo_Global.vi" "File Index"(w18) -> ()
      n6 = call "IMAQ Create"("Image Name"="Camera Name", "Image Type"=w13) -> ("New Image"=w16:T8, "error out"=w14:errorcluster)  [unwired: 2 in, 1 out]
      n7 = local write "stop"(FALSE ("stop")) -> ()
      "Status" <- "Initializing..."
    }
    frame #1 {
      n8 = case shown="True" w21 {
        tunnel: w28 -> [_ w34]
        tunnel: w27 -> [w29 w35]
        tunnel: w26 -> [_ w47]
        tunnel: [w29 w44] -> w22
        frame False {
        }
        frame True {
          w50 = FALSE  # Debug?
          n9 = call "Setup For Triggered Images USB3 v4.4.vi"("error in"=w35, "Timeout"="Timeout (ms)", "Gain"="Gain", "Shutter speed"="Shutter speed", "Camera Name"=w34) -> ("Error out"=w38:errorcluster, "Session Out"=w39:T2, "Height"=w37:u32, "Width"=w36:u32, "DeviceID"=w30:string)
          n10 = case shown="True" w50 {
            tunnel: [w51 w55] -> w49
            tunnel: [w52 w54] -> w48
            tunnel: w39 -> [w51 w56]
            tunnel: w38 -> [w52 w53]
            frame False {
            }
            frame True {
              n11 = call "CheckCameraAttributes-USB3.vi"("error in"=w53, "Camera Name"=w56) -> ("error out"=w54:errorcluster, "Session Out"=w55:T2)
            }
          }
          n12 = call "GetStatusInfo.vi"("error in"=w48, "Camera In"=w49) -> ("Status Info"=w46:T9, "error out"=w43:errorcluster, "Camera Out"=w42:T2)  [unwired: 1 in]
          n13 = while {
            tunnel: w42 -> [w67]
            tunnel: w47 -> [w66]
            tunnel: w37 -> [w65]
            tunnel: w36 -> [w64]
            tunnel: w46 -> [w63]
            tunnel: [w62] -> w41
            shift-right: [0] -> _
            shift-left: 0 -> [w61]
            shift-right: [w58] -> w40
            shift-left: w43 -> [w59]
            tunnel: w30 -> [w57]
            i -> [w69]
            stop <- w68 stop-if-true
            n14 = stacked-sequence {
              seq-local: [_ _ _ w184 _ _ _ _] -> [_ _ _ _ _ w258 _ _]
              seq-local: [_ _ _ _ _ w254 _ _] -> [_ _ _ _ _ _ _ w268]
              seq-local: [_ w89 _ _ _ _ _ _] -> [_ _ w158 _ _ _ _ _]
              seq-local: [_ _ w157 _ _ _ _ _] -> [_ _ _ w175 _ _ _ _]
              tunnel: [_ _ _ _ _ _ _ "stop"] -> w68
              tunnel: w67 -> [_ w81 _ _ _ _ _ _]
              tunnel: w66 -> [_ w97 _ _ _ _ _ _]
              tunnel: w65 -> [_ w96 _ _ _ _ _ _]
              tunnel: w64 -> [_ w95 _ _ _ _ _ _]
              tunnel: w63 -> [_ w93 _ _ _ _ _ _]
              tunnel: [_ w76 _ _ _ _ _ _] -> w62
              tunnel: [_ w75 _ _ _ _ _ _] -> w58
              tunnel: w61 -> [_ w92 _ _ _ _ _ _]
              tunnel: w59 -> [_ w84 _ _ _ _ _ _]
              tunnel: w57 -> [_ _ _ _ w205 _ _ _]
              frame #0 {
                n15 = local read "Send Flea data to Igor?"() -> (w70:bool)